vi "TLB Native Dynamic Events ver 0.25.vi"() -> ()   [LabVIEW 2018] (continued)
                }
              }
            }
          }
          frame 18 {
            # ">>> Motor control cluster >>>"
            # ">>> yStepper command>>>"
            # ">> Manual override >>"
            n401 = Equal?(x=w1065, y=u8 60) -> (x = y?=w1063:bool)
            n402 = Dequeue Element(queue=w1075, timeout in ms (-1)=w1074, error in (no error)=w1073) -> (element=w1072:T8)  [unwired: 3 out]
            n403 = case shown="\"Start Task 1\", Default" w1072 {
              tunnel: [w1084 State_Type_Definitions,_for_0.26g_versions_and_later_2."True Stop" ("Enum")] -> w1077
              tunnel: [w1087 w1104] -> w1070
              tunnel: [State_Type_Definitions,_for_0.26g_versions_and_later_2."Idle" ("Enum") State_Type_Definitions,_for_0.26g_versions_and_later_2."Shutdown" ("Enum")] -> w1069
              tunnel: w1071 -> [w1078 _]
              tunnel: w1076 -> [w1083 w1101]
              tunnel: w1063 -> [w1082 _]
              frame "Start Task 1", Default {
                # ">> Is time up? >>"
                # "Determines if object is in range to pick up"
                # ">> Manual override >>"
                n404 = case shown="True" w1082 {
                  tunnel: [w1091 w1097] -> w1087
                  tunnel: w1083 -> [w1089 w1095]
                  frame False {
                    n405 = for {
                      tunnel: string[] ["Z STEPPER CAM HEIGHT", "READ STEPPER VALUES"] ("element") -> [w1092] mode=indexing
                      shift-right: [w1094] -> w1091
                      shift-left: w1089 -> [w1093]
                      n406 = Enqueue Element(queue=w1093, element=w1092) -> (queue out=w1094:refnum<queue>)  [unwired: 2 in, 2 out]
                    }
                  }
                  frame True {
                    n407 = for {
                      shift-right: [w1099] -> w1097
                      shift-left: w1095 -> [w1100]
                      tunnel: string[] ["SET TIMER 5", "", ""] -> [w1098] mode=indexing
                      n408 = Enqueue Element(queue=w1100, element=w1098) -> (queue out=w1099:refnum<queue>)  [unwired: 2 in, 2 out]
                    }
                  }
                }
                n409 = Or(x=w1082, y=w1078) -> (x .or. y?=w1085:bool)
                n410 = Select(t=State_Type_Definitions,_for_0.26g_versions_and_later_2."True Stop" ("Enum"), s=w1078, f=State_Type_Definitions,_for_0.26g_versions_and_later_2."Task 5D" ("Enum")) -> (s? t:f=w1080:T16)
                n411 = Select(t=w1080, s=w1085, f=State_Type_Definitions,_for_0.26g_versions_and_later_2."Task 5C" ("Enum")) -> (s? t:f=w1084:T16)
              }
              frame "Exit" {
                n412 = for {
                  shift-right: [w1107] -> w1104
                  shift-left: w1101 -> [w1108]
                  tunnel: string[] ["STOP", "RESET ENCODERS", "RESET YAW", "ARDUINO MODE 0"] -> [w1106] mode=indexing
                  n413 = Enqueue Element(queue=w1108, element=w1106) -> (queue out=w1107:refnum<queue>)  [unwired: 2 in, 2 out]
                }
              }
            }
          }
          frame 19 {
            # ">>> yStepper command>>>"
            n414 = Dequeue Element(queue=w1116, timeout in ms (-1)=w1115, error in (no error)=w1114) -> (element=w1113:T8)  [unwired: 3 out]
            n415 = case shown="\"Start Task 1\", Default" w1113 {
              tunnel: [w1128 State_Type_Definitions,_for_0.26g_versions_and_later_2."True Stop" ("Enum")] -> w1120
              tunnel: [w1131 w1148] -> w1119
              tunnel: [State_Type_Definitions,_for_0.26g_versions_and_later_2."Idle" ("Enum") State_Type_Definitions,_for_0.26g_versions_and_later_2."Shutdown" ("Enum")] -> w1121
              tunnel: w1117 -> [w1127 _]
              tunnel: w1118 -> [w1123 w1145]
              tunnel: w1111 -> [w1122 _]
              frame "Start Task 1", Default {
                # ">> T: Breaks out of state loop; F: Stays in loop>>"
                # ">> Manual override >>"
                # ">> Checks if time is up>>"
                # "Stays in Task 5D until the object is detected"
                # "T: Go back to idle, F: Continue with task\""
                # ">> Manual override >>"
                n416 = case shown="False" w1122 {
                  tunnel: [w1135 w1141] -> w1131
                  tunnel: w1123 -> [w1133 w1139]
                  frame False {
                    n417 = for {
                      tunnel: string[] ["START TIMER", "OPEN CLAW", ""] ("element") -> [w1136] mode=indexing
                      shift-right: [w1138] -> w1135
                      shift-left: w1133 -> [w1137]
                      n418 = Enqueue Element(queue=w1137, element=w1136) -> (queue out=w1138:refnum<queue>)  [unwired: 2 in, 2 out]
                    }
                  }
                  frame True {
                    n419 = for {
                      shift-right: [w1143] -> w1141
                      shift-left: w1139 -> [w1144]
                      tunnel: string[] ["CAM CLOSE", "", ""] -> [w1142] mode=indexing
                      n420 = Enqueue Element(queue=w1144, element=w1142) -> (queue out=w1143:refnum<queue>)  [unwired: 2 in, 2 out]
                    }
                  }
                }
                n421 = Or(x=w1122, y=w1127) -> (x .or. y?=w1129:bool)
                n422 = Select(t=State_Type_Definitions,_for_0.26g_versions_and_later_2."True Stop" ("Enum"), s=w1127, f=State_Type_Definitions,_for_0.26g_versions_and_later_2."True Stop" ("Enum")) -> (s? t:f=w1124:T16)
                n423 = Select(t=w1124, s=w1129, f=State_Type_Definitions,_for_0.26g_versions_and_later_2."Task 5D" ("Enum")) -> (s? t:f=w1128:T16)
              }
              frame "Exit" {
                n424 = for {
                  shift-right: [w1151] -> w1148
                  shift-left: w1145 -> [w1152]
                  tunnel: string[] ["STOP", "RESET ENCODERS", "RESET YAW", "ARDUINO MODE 0"] -> [w1150] mode=indexing
                  n425 = Enqueue Element(queue=w1152, element=w1150) -> (queue out=w1151:refnum<queue>)  [unwired: 2 in, 2 out]
                }
              }
            }
          }
          frame 20 {
            # ">>> yStepper command>>>"
            n426 = Dequeue Element(queue=w1166, timeout in ms (-1)=w1167, error in (no error)=w1168) -> (element=w1170:T8)  [unwired: 3 out]
            n427 = formula code="if (pos < 100)\ny = 41;\n\nelse if (pos >= 100 && pos <= 140)\ny = 30;\n\nelse if (pos >= 141 && pos <= 170)\ny = 25;\n\nelse if (pos >= 171 &&pos <= 180) \ny = 20;\n\nelse if (pos >= 181&& pos <= 200)\ny = 15;\n\nelse if (pos >= 201 && pos <= 230)\ny = 10;\n\nelse if (pos >= 231 && pos <= 320)\ny = 8;\n\nelse if (pos > 320)\ny = 0;"("pos"=w1158) -> ("y"=w1161:dbl)
            n428 = To Unsigned Byte Integer(number=w1161) -> (unsigned 8bit integer=w1156:u8)
            n429 = Equal?(x=w1157, y=w1156) -> (x = y?=w1155:bool)
            n430 = case shown="\"Start Task 1\", Default" w1170 {
              tunnel: [w1177 State_Type_Definitions,_for_0.26g_versions_and_later_2."True Stop" ("Enum")] -> w1164
              tunnel: [w1180 w1197] -> w1162
              tunnel: [State_Type_Definitions,_for_0.26g_versions_and_later_2."Idle" ("Enum") State_Type_Definitions,_for_0.26g_versions_and_later_2."Shutdown" ("Enum")] -> w1163
              tunnel: w1169 -> [w1176 _]
              tunnel: w1165 -> [w1172 w1194]
              tunnel: w1155 -> [w1171 _]
              frame "Start Task 1", Default {
                # ">> T: Breaks out of state loop; F: Stays in loop>>"
                # ">> Manual override >>"
                # ">> Checks if time is up>>"
                # "Stays in Task 5D until the object is detected"
                # "T: Go back to idle, F: Continue with task\""
                # ">> Manual override >>"
                n431 = case shown="False" w1171 {
                  tunnel: [w1184 w1190] -> w1180
                  tunnel: w1172 -> [w1182 w1188]
                  frame False {
                    n432 = for {
                      tunnel: string[] ["READ STEPPER VALUES", "Y STEPPER CONTROL", ""] ("element") -> [w1185] mode=indexing
                      shift-right: [w1187] -> w1184
                      shift-left: w1182 -> [w1186]
                      n433 = Enqueue Element(queue=w1186, element=w1185) -> (queue out=w1187:refnum<queue>)  [unwired: 2 in, 2 out]
                    }
                  }
                  frame True {
                    n434 = for {
                      shift-right: [w1192] -> w1190
                      shift-left: w1188 -> [w1193]
                      tunnel: string[] ["CAM CLOSE", "DISPOSE BUFFERS", ""] -> [w1191] mode=indexing
                      n435 = Enqueue Element(queue=w1193, element=w1191) -> (queue out=w1192:refnum<queue>)  [unwired: 2 in, 2 out]
                    }
                  }
                }
                n436 = Or(x=w1171, y=w1176) -> (x .or. y?=w1178:bool)
                n437 = Select(t=State_Type_Definitions,_for_0.26g_versions_and_later_2."True Stop" ("Enum"), s=w1176, f=State_Type_Definitions,_for_0.26g_versions_and_later_2."Task 5F: ARM GRAB HEIGHT" ("Enum")) -> (s? t:f=w1173:T16)
                n438 = Select(t=w1173, s=w1178, f=State_Type_Definitions,_for_0.26g_versions_and_later_2."Task 5E: POSITION ARM" ("Enum")) -> (s? t:f=w1177:T16)
              }
              frame "Exit" {
                n439 = for {
                  shift-right: [w1200] -> w1197
                  shift-left: w1194 -> [w1201]
                  tunnel: string[] ["STOP", "RESET ENCODERS", "RESET YAW", "ARDUINO MODE 0"] -> [w1199] mode=indexing
                  n440 = Enqueue Element(queue=w1201, element=w1199) -> (queue out=w1200:refnum<queue>)  [unwired: 2 in, 2 out]
                }
              }
            }
            n441 = Bundle By Name(cluster=w1160, "yStepper desired"=w1156) -> (w1159:T18)
          }
          frame 21 {
            # ">>> Motor control cluster >>>"
            # ">>> yStepper command>>>"
            # ">> Manual override >>"
            n442 = Dequeue Element(queue=w1212, timeout in ms (-1)=w1211, error in (no error)=w1213) -> (element=w1210:T8)  [unwired: 3 out]
            n443 = Equal?(x=w1209, y=u8 1) -> (x = y?=w1207:bool)
            n444 = case shown="\"Start Task 1\", Default" w1210 {
              tunnel: [w1223 State_Type_Definitions,_for_0.26g_versions_and_later_2."True Stop" ("Enum")] -> w1214
              tunnel: [w1226 w1243] -> w1215
              tunnel: [State_Type_Definitions,_for_0.26g_versions_and_later_2."Idle" ("Enum") State_Type_Definitions,_for_0.26g_versions_and_later_2."Shutdown" ("Enum")] -> w1216
              tunnel: w1207 -> [w1222 _]
              tunnel: w1206 -> [w1221 _]
              tunnel: w1205 -> [w1217 w1240]
              frame "Start Task 1", Default {
                # "Stays in Task 5F until stepper reaches desired \nheight"
                # "T: Go back to idle, F: Continue with task\""
                # ">> Manual override >>"
                n445 = case shown="True" w1222 {
                  tunnel: [w1230 w1236] -> w1226
                  tunnel: w1217 -> [w1228 w1234]
                  frame False {
                    n446 = for {
                      tunnel: string[] ["Z STEPPER GRAB HEIGHT", "READ STEPPER VALUES"] ("element") -> [w1231] mode=indexing
                      shift-right: [w1233] -> w1230
                      shift-left: w1228 -> [w1232]
                      n447 = Enqueue Element(queue=w1232, element=w1231) -> (queue out=w1233:refnum<queue>)  [unwired: 2 in, 2 out]
                    }
                  }
                  frame True {
                    n448 = for {
                      shift-right: [w1238] -> w1236
                      shift-left: w1234 -> [w1239]
                      tunnel: string[] ["SET TIMER 5", "CLOSE CLAW", ""] -> [w1237] mode=indexing
                      n449 = Enqueue Element(queue=w1239, element=w1237) -> (queue out=w1238:refnum<queue>)  [unwired: 2 in, 2 out]
                    }
                  }
                }
                n450 = Or(x=w1222, y=w1221) -> (x .or. y?=w1224:bool)
                n451 = Select(t=State_Type_Definitions,_for_0.26g_versions_and_later_2."True Stop" ("Enum"), s=w1221, f=State_Type_Definitions,_for_0.26g_versions_and_later_2."Task 5G: CLOSE CLAW" ("Enum")) -> (s? t:f=w1218:T16)
                n452 = Select(t=w1218, s=w1224, f=State_Type_Definitions,_for_0.26g_versions_and_later_2."Task 5F: ARM GRAB HEIGHT" ("Enum")) -> (s? t:f=w1223:T16)
              }
              frame "Exit" {
                n453 = for {
                  shift-right: [w1246] -> w1243
                  shift-left: w1240 -> [w1247]
                  tunnel: string[] ["STOP", "RESET ENCODERS", "RESET YAW", "ARDUINO MODE 0"] -> [w1245] mode=indexing
                  n454 = Enqueue Element(queue=w1247, element=w1245) -> (queue out=w1246:refnum<queue>)  [unwired: 2 in, 2 out]
                }
              }
            }
          }
          frame 22 {
            # ">>> yStepper command>>>"
            # ">> Manual override >>"
            n455 = Dequeue Element(queue=w1258, timeout in ms (-1)=w1257, error in (no error)=w1256) -> (element=w1255:T8)  [unwired: 3 out]
            n456 = case shown="\"Start Task 1\", Default" w1255 {
              tunnel: [w1267 State_Type_Definitions,_for_0.26g_versions_and_later_2."True Stop" ("Enum")] -> w1260
              tunnel: [w1270 w1287] -> w1253
              tunnel: [State_Type_Definitions,_for_0.26g_versions_and_later_2."Idle" ("Enum") State_Type_Definitions,_for_0.26g_versions_and_later_2."Shutdown" ("Enum")] -> w1252
              tunnel: w1254 -> [w1261 _]
              tunnel: w1259 -> [w1266 w1284]
              tunnel: w1250 -> [w1265 _]
              frame "Start Task 1", Default {
                # ">> Is time up? >>"
                # "Determines if object is in range to pick up"
                # ">> Manual override >>"
                n457 = case shown="True" w1265 {
                  tunnel: [w1274 w1280] -> w1270
                  tunnel: w1266 -> [w1272 w1278]
                  frame False {
                    n458 = for {
                      tunnel: string[] ["CLOSE CLAW", "START TIMER"] ("element") -> [w1275] mode=indexing
                      shift-right: [w1277] -> w1274
                      shift-left: w1272 -> [w1276]
                      n459 = Enqueue Element(queue=w1276, element=w1275) -> (queue out=w1277:refnum<queue>)  [unwired: 2 in, 2 out]
                    }
                  }
                  frame True {
                    n460 = for {
                      shift-right: [w1282] -> w1280
                      shift-left: w1278 -> [w1283]
                      tunnel: string[] ["READ STEPPER VALUES", "", ""] -> [w1281] mode=indexing
                      n461 = Enqueue Element(queue=w1283, element=w1281) -> (queue out=w1282:refnum<queue>)  [unwired: 2 in, 2 out]
                    }
                  }
                }
                n462 = Or(x=w1265, y=w1261) -> (x .or. y?=w1268:bool)
                n463 = Select(t=State_Type_Definitions,_for_0.26g_versions_and_later_2."True Stop" ("Enum"), s=w1261, f=State_Type_Definitions,_for_0.26g_versions_and_later_2."Task 5H: RAISE ARM" ("Enum")) -> (s? t:f=w1263:T16)
                n464 = Select(t=w1263, s=w1268, f=State_Type_Definitions,_for_0.26g_versions_and_later_2."Task 5G: CLOSE CLAW" ("Enum")) -> (s? t:f=w1267:T16)
              }
              frame "Exit" {
                n465 = for {
                  shift-right: [w1290] -> w1287
                  shift-left: w1284 -> [w1291]
                  tunnel: string[] ["STOP", "RESET ENCODERS", "RESET YAW", "ARDUINO MODE 0"] -> [w1289] mode=indexing
                  n466 = Enqueue Element(queue=w1291, element=w1289) -> (queue out=w1290:refnum<queue>)  [unwired: 2 in, 2 out]
                }
              }
            }
          }
          frame 23 {
            # ">>> yStepper command>>>"
            # ">> Manual override >>"
            n467 = Dequeue Element(queue=w1302, timeout in ms (-1)=w1301, error in (no error)=w1303) -> (element=w1300:T8)  [unwired: 3 out]
            n468 = Equal?(x=w1299, y=u8 60) -> (x = y?=w1297:bool)
            n469 = case shown="\"Start Task 1\", Default" w1300 {
              tunnel: [w1313 State_Type_Definitions,_for_0.26g_versions_and_later_2."True Stop" ("Enum")] -> w1304
              tunnel: [w1316 w1333] -> w1305
              tunnel: [State_Type_Definitions,_for_0.26g_versions_and_later_2."Idle" ("Enum") State_Type_Definitions,_for_0.26g_versions_and_later_2."Shutdown" ("Enum")] -> w1306
              tunnel: w1297 -> [w1312 _]
              tunnel: w1296 -> [w1311 _]
              tunnel: w1295 -> [w1307 w1330]
              frame "Start Task 1", Default {
                # "Stays in Task 5_A until stepper reaches desired \nheight"
                # "T: Go back to idle, F: Continue with task\""
                # ">> Manual override >>"
                n470 = case shown="False" w1312 {
                  tunnel: [w1320 w1326] -> w1316
                  tunnel: w1307 -> [w1318 w1324]
                  frame False {
                    n471 = for {
                      tunnel: string[] ["Z STEPPER CAM HEIGHT", "READ STEPPER VALUES"] ("element") -> [w1321] mode=indexing
                      shift-right: [w1323] -> w1320
                      shift-left: w1318 -> [w1322]
                      n472 = Enqueue Element(queue=w1322, element=w1321) -> (queue out=w1323:refnum<queue>)  [unwired: 2 in, 2 out]
                    }
                  }
                  frame True {
                    n473 = for {
                      shift-right: [w1328] -> w1326
                      shift-left: w1324 -> [w1329]
                      tunnel: string[] ["ARDUINO - ULTRASONIC", "READ ULTRASONIC", ""] -> [w1327] mode=indexing
                      n474 = Enqueue Element(queue=w1329, element=w1327) -> (queue out=w1328:refnum<queue>)  [unwired: 2 in, 2 out]
                    }
                  }
                }
                n475 = Or(x=w1312, y=w1311) -> (x .or. y?=w1314:bool)
                n476 = Select(t=State_Type_Definitions,_for_0.26g_versions_and_later_2."True Stop" ("Enum"), s=w1311, f=State_Type_Definitions,_for_0.26g_versions_and_later_2."True Stop" ("Enum")) -> (s? t:f=w1308:T16)
                n477 = Select(t=w1308, s=w1314, f=State_Type_Definitions,_for_0.26g_versions_and_later_2."Task 5H: RAISE ARM" ("Enum")) -> (s? t:f=w1313:T16)
              }
              frame "Exit" {
                n478 = for {
                  shift-right: [w1336] -> w1333
                  shift-left: w1330 -> [w1337]
                  tunnel: string[] ["STOP", "RESET ENCODERS", "RESET YAW", "ARDUINO MODE 0"] -> [w1335] mode=indexing
                  n479 = Enqueue Element(queue=w1337, element=w1335) -> (queue out=w1336:refnum<queue>)  [unwired: 2 in, 2 out]
                }
              }
            }
          }
          frame 24 {
            # ">>> yStepper command>>>"
            n480 = Dequeue Element(queue=w1347, timeout in ms (-1)=w1346, error in (no error)=w1345) -> (element=w1352:T8)  [unwired: 3 out]
            n481 = Equal?(x=w1343, y=u8 60) -> (x = y?=w1342:bool)
            n482 = case shown="\"Start Task 1\", Default" w1352 {
              tunnel: [w1359 State_Type_Definitions,_for_0.26g_versions_and_later_2."True Stop" ("Enum")] -> w1350
              tunnel: [w1358 w1376] -> w1349
              tunnel: [State_Type_Definitions,_for_0.26g_versions_and_later_2."Idle" ("Enum") State_Type_Definitions,_for_0.26g_versions_and_later_2."Shutdown" ("Enum")] -> w1351
              tunnel: w1348 -> [w1354 _]
              tunnel: w1344 -> [w1356 _]
              tunnel: w1342 -> [w1353 _]
              frame "Start Task 1", Default {
                n483 = case shown="False" w1353 {
                  tunnel: [w1364 w1370] -> w1358
                  tunnel: w1356 -> [w1362 w1368]
                  frame False {
                    n484 = for {
                      tunnel: string[] ["Z STEPPER CAM HEIGHT", "READ STEPPER VALUES"] ("element") -> [w1365] mode=indexing
                      shift-right: [w1367] -> w1364
                      shift-left: w1362 -> [w1366]
                      n485 = Enqueue Element(queue=w1366, element=w1365) -> (queue out=w1367:refnum<queue>)  [unwired: 2 in, 2 out]
                    }
                  }
                  frame True {
                    n486 = for {
                      shift-right: [w1372] -> w1370
                      shift-left: w1368 -> [w1373]
                      tunnel: string[] ["CAM ACQ", "OPEN LOG CAM"] -> [w1371] mode=indexing
                      n487 = Enqueue Element(queue=w1373, element=w1371) -> (queue out=w1372:refnum<queue>)  [unwired: 2 in, 2 out]
                    }
                  }
                }
                n488 = Or(x=w1353, y=w1354) -> (x .or. y?=w1355:bool)
                n489 = Select(t=State_Type_Definitions,_for_0.26g_versions_and_later_2."Task 6_B" ("Enum"), s=w1355, f=State_Type_Definitions,_for_0.26g_versions_and_later_2."Task 6_A" ("Enum")) -> (s? t:f=w1359:T16)
              }
              frame "Exit" {
                n490 = for {
                  shift-right: [w1379] -> w1376
                  shift-left: _ -> [w1380]
                  tunnel: string[] ["STOP", "RESET ENCODERS", "RESET YAW", "ARDUINO MODE 0"] -> [w1378] mode=indexing
                  n491 = Enqueue Element(queue=w1380, element=w1378) -> (queue out=w1379:refnum<queue>)  [unwired: 2 in, 2 out]
                }
              }
            }
          }
          frame 25 {
            # ">>> yStepper command>>>"
            n492 = Dequeue Element(queue=w1392, timeout in ms (-1)=w1390, error in (no error)=w1391) -> (element=w1389:T8)  [unwired: 3 out]
            n493 = case shown="\"Start Task 1\", Default" w1389 {
              tunnel: [w1399 State_Type_Definitions,_for_0.26g_versions_and_later_2."True Stop" ("Enum")] -> w1385
              tunnel: [w1398 w1417] -> w1393
              tunnel: [State_Type_Definitions,_for_0.26g_versions_and_later_2."Idle" ("Enum") State_Type_Definitions,_for_0.26g_versions_and_later_2."Shutdown" ("Enum")] -> w1386
              tunnel: w1388 -> [w1394 _]
              tunnel: w1387 -> [w1396 _]
              tunnel: w1384 -> [w1395 w1414]
              frame "Start Task 1", Default {
                # ">> Manual override >>"
                n494 = case shown="False" w1396 {
                  tunnel: [w1404 w1410] -> w1398
                  tunnel: w1395 -> [w1403 w1408]
                  frame False {
                    n495 = for {
                      shift-right: [w1407] -> w1404
                      shift-left: w1403 -> [w1406]
                      tunnel: string[] ["CAM ACQ", "PROCESS IMAGE", "OPEN CLAW"] -> [w1405] mode=indexing
                      n496 = Enqueue Element(queue=w1406, element=w1405) -> (queue out=w1407:refnum<queue>)  [unwired: 2 in, 2 out]
                    }
                  }
                  frame True {
                    n497 = for {
                      shift-right: [w1412] -> w1410
                      shift-left: w1408 -> [w1413]
                      tunnel: string[] ["CAM ACQ", "PROCESS IMAGE", "CLOSE CLAW"] -> [w1411] mode=indexing
                      n498 = Enqueue Element(queue=w1413, element=w1411) -> (queue out=w1412:refnum<queue>)  [unwired: 2 in, 2 out]
                    }
                  }
                }
                n499 = Select(t=State_Type_Definitions,_for_0.26g_versions_and_later_2."True Stop" ("Enum"), s=w1394, f=State_Type_Definitions,_for_0.26g_versions_and_later_2."Task 6_B" ("Enum")) -> (s? t:f=w1399:T16)
              }
              frame "Exit" {
                # ">> State after true stop >>"
                # ">> Goes to true stop >>"
                n500 = for {
                  shift-right: [w1420] -> w1417
                  shift-left: w1414 -> [w1421]
                  tunnel: string[] ["STOP", "RESET ENCODERS", "RESET YAW", ""] -> [w1419] mode=indexing
                  n501 = Enqueue Element(queue=w1421, element=w1419) -> (queue out=w1420:refnum<queue>)  [unwired: 2 in, 2 out]
                }
              }
            }
          }
          frame 26 {
          }
          frame 27 {
            # ">>> Motor control cluster >>>"
            # ">>> yStepper command>>>"
            # ">> Manual override >>"
            n502 = Dequeue Element(queue=w1438, timeout in ms (-1)=w1437, error in (no error)=w1439) -> (element=w1436:T8)  [unwired: 3 out]
            n503 = Equal?(x=w1435, y=u8 60) -> (x = y?=w1433:bool)
            n504 = case shown="\"Start Task 1\", Default" w1436 {
              tunnel: [w1449 State_Type_Definitions,_for_0.26g_versions_and_later_2."True Stop" ("Enum")] -> w1440
              tunnel: [w1452 w1469] -> w1441
              tunnel: [State_Type_Definitions,_for_0.26g_versions_and_later_2."Idle" ("Enum") State_Type_Definitions,_for_0.26g_versions_and_later_2."Shutdown" ("Enum")] -> w1442
              tunnel: w1433 -> [w1448 _]
              tunnel: w1432 -> [w1447 _]
              tunnel: w1431 -> [w1443 w1466]
              frame "Start Task 1", Default {
                # "Stays in Task 5_A until stepper reaches desired \nheight"
                # "T: Go back to idle, F: Continue with task\""
                # ">> Manual override >>"
                n505 = case shown="False" w1448 {
                  tunnel: [w1456 w1462] -> w1452
                  tunnel: w1443 -> [w1454 w1460]
                  frame False {
                    n506 = for {
                      tunnel: string[] ["Z STEPPER CAM HEIGHT", "READ STEPPER VALUES"] ("element") -> [w1457] mode=indexing
                      shift-right: [w1459] -> w1456
                      shift-left: w1454 -> [w1458]
                      n507 = Enqueue Element(queue=w1458, element=w1457) -> (queue out=w1459:refnum<queue>)  [unwired: 2 in, 2 out]
                    }
                  }
                  frame True {
                    n508 = for {
                      shift-right: [w1464] -> w1462
                      shift-left: w1460 -> [w1465]
                      tunnel: string[] ["ARDUINO - ULTRASONIC", "READ ULTRASONIC", ""] -> [w1463] mode=indexing
                      n509 = Enqueue Element(queue=w1465, element=w1463) -> (queue out=w1464:refnum<queue>)  [unwired: 2 in, 2 out]
                    }
                  }
                }
                n510 = Or(x=w1448, y=w1447) -> (x .or. y?=w1450:bool)
                n511 = Select(t=State_Type_Definitions,_for_0.26g_versions_and_later_2."True Stop" ("Enum"), s=w1447, f=State_Type_Definitions,_for_0.26g_versions_and_later_2."Task 8B: MOVE TO BOX" ("Enum")) -> (s? t:f=w1444:T16)
                n512 = Select(t=w1444, s=w1450, f=State_Type_Definitions,_for_0.26g_versions_and_later_2."Task 8A: RAISE ARM" ("Enum")) -> (s? t:f=w1449:T16)
              }
              frame "Exit" {
                n513 = for {
                  shift-right: [w1472] -> w1469
                  shift-left: w1466 -> [w1473]
                  tunnel: string[] ["STOP", "RESET ENCODERS", "RESET YAW", "ARDUINO MODE 0"] -> [w1471] mode=indexing
                  n514 = Enqueue Element(queue=w1473, element=w1471) -> (queue out=w1472:refnum<queue>)  [unwired: 2 in, 2 out]
                }
              }
            }
          }
          frame 28 {
            w1481 = u8 15 ("y")
            # ">>> yStepper command>>>"
            n515 = Less?(x=w1478, y=w1481) -> (x < y?=w1479:bool)
            n516 = Dequeue Element(queue=w1485, timeout in ms (-1)=w1484, error in (no error)=w1486) -> (element=w1483:T8)  [unwired: 3 out]
            n517 = Less?(x=w1477, y=w1481) -> (x < y?=w1480:bool)
            n518 = And(x=w1480, y=w1479) -> (x .and. y?=w1476:bool)
            n519 = case shown="\"Start Task 1\", Default" w1483 {
              tunnel: [w1498 State_Type_Definitions,_for_0.26g_versions_and_later_2."True Stop" ("Enum")] -> w1488
              tunnel: [w1501 w1518] -> w1487
              tunnel: [State_Type_Definitions,_for_0.26g_versions_and_later_2."Idle" ("Enum") State_Type_Definitions,_for_0.26g_versions_and_later_2."Shutdown" ("Enum")] -> w1489
              tunnel: w1491 -> [w1497 _]
              tunnel: w1490 -> [w1493 w1515]
              tunnel: w1476 -> [w1492 _]
              frame "Start Task 1", Default {
                # "Stays in Task 5_B to capture image over 5 seconds"
                # "T: Go back to idle, F: Continue with task\""
                # ">> Manual override >>"
                n520 = case shown="True" w1492 {
                  tunnel: [w1505 w1511] -> w1501
                  tunnel: w1493 -> [w1503 w1509]
                  frame False {
                    n521 = for {
                      tunnel: string[] ["FORWARD", "READ ULTRASONIC", "READ NAVX"] ("element") -> [w1506] mode=indexing
                      shift-right: [w1508] -> w1505
                      shift-left: w1503 -> [w1507]
                      n522 = Enqueue Element(queue=w1507, element=w1506) -> (queue out=w1508:refnum<queue>)  [unwired: 2 in, 2 out]
                    }
                  }
                  frame True {
                    n523 = for {
                      shift-right: [w1513] -> w1511
                      shift-left: w1509 -> [w1514]
                      tunnel: string[] ["STOP", "RESET ENCODERS", "OPEN LOG CAM", "SET TIMER 2", "OPEN IMAQ REF"] -> [w1512] mode=indexing
                      n524 = Enqueue Element(queue=w1514, element=w1512) -> (queue out=w1513:refnum<queue>)  [unwired: 2 in, 2 out]
                    }
                  }
                }
                n525 = Or(x=w1492, y=w1497) -> (x .or. y?=w1499:bool)
                n526 = Select(t=State_Type_Definitions,_for_0.26g_versions_and_later_2."True Stop" ("Enum"), s=w1497, f=State_Type_Definitions,_for_0.26g_versions_and_later_2."Task 8C: CAM BURST" ("Enum")) -> (s? t:f=w1494:T16)
                n527 = Select(t=w1494, s=w1499, f=State_Type_Definitions,_for_0.26g_versions_and_later_2."Task 8B: MOVE TO BOX" ("Enum")) -> (s? t:f=w1498:T16)
              }
              frame "Exit" {
                n528 = for {
                  shift-right: [w1521] -> w1518
                  shift-left: w1515 -> [w1522]
                  tunnel: string[] ["STOP", "RESET ENCODERS", "RESET YAW", "ARDUINO MODE 0"] -> [w1520] mode=indexing
                  n529 = Enqueue Element(queue=w1522, element=w1520) -> (queue out=w1521:refnum<queue>)  [unwired: 2 in, 2 out]
                }
              }
            }
          }
          frame 29 {
            # ">>> Motor control cluster >>>"
            # ">>> yStepper command>>>"
            # ">> Manual override >>"
            n530 = Dequeue Element(queue=w1533, timeout in ms (-1)=w1532, error in (no error)=w1531) -> (element=w1530:T8)  [unwired: 3 out]
            n531 = case shown="\"Start Task 1\", Default" w1530 {
              tunnel: [w1542 State_Type_Definitions,_for_0.26g_versions_and_later_2."True Stop" ("Enum")] -> w1535
              tunnel: [w1545 w1562] -> w1528
              tunnel: [State_Type_Definitions,_for_0.26g_versions_and_later_2."Idle" ("Enum") State_Type_Definitions,_for_0.26g_versions_and_later_2."Shutdown" ("Enum")] -> w1527
              tunnel: w1529 -> [w1536 _]
              tunnel: w1534 -> [w1541 w1559]
              tunnel: w1525 -> [w1540 _]
              frame "Start Task 1", Default {
                # ">> Is time up? >>"
                # "Determines if object is in range to pick up"
                # ">> Manual override >>"
                n532 = case shown="True" w1540 {
                  tunnel: [w1549 w1555] -> w1545
                  tunnel: w1541 -> [w1547 w1553]
                  frame False {
                    n533 = for {
                      tunnel: string[] ["CAM ACQ", "START TIMER"] ("element") -> [w1550] mode=indexing
                      shift-right: [w1552] -> w1549
                      shift-left: w1547 -> [w1551]
                      n534 = Enqueue Element(queue=w1551, element=w1550) -> (queue out=w1552:refnum<queue>)  [unwired: 2 in, 2 out]
                    }
                  }
                  frame True {
                    n535 = for {
                      shift-right: [w1557] -> w1555
                      shift-left: w1553 -> [w1558]
                      tunnel: string[] ["CAM CLOSE", "PROCESS IMAGE", "SET TIMER 5"] -> [w1556] mode=indexing
                      n536 = Enqueue Element(queue=w1558, element=w1556) -> (queue out=w1557:refnum<queue>)  [unwired: 2 in, 2 out]
                    }
                  }
                }
                n537 = Or(x=w1540, y=w1536) -> (x .or. y?=w1543:bool)
                n538 = Select(t=State_Type_Definitions,_for_0.26g_versions_and_later_2."True Stop" ("Enum"), s=w1536, f=State_Type_Definitions,_for_0.26g_versions_and_later_2."Task 8D: PROCESS IMAGE" ("Enum")) -> (s? t:f=w1538:T16)
                n539 = Select(t=w1538, s=w1543, f=State_Type_Definitions,_for_0.26g_versions_and_later_2."Task 8C: CAM BURST" ("Enum")) -> (s? t:f=w1542:T16)
              }
              frame "Exit" {
                n540 = for {
                  shift-right: [w1565] -> w1562
                  shift-left: w1559 -> [w1566]
                  tunnel: string[] ["STOP", "RESET ENCODERS", "RESET YAW", "ARDUINO MODE 0"] -> [w1564] mode=indexing
                  n541 = Enqueue Element(queue=w1566, element=w1564) -> (queue out=w1565:refnum<queue>)  [unwired: 2 in, 2 out]
                }
              }
            }
          }
          frame 30 {
            # ">>> yStepper command>>>"
            n542 = Dequeue Element(queue=w1574, timeout in ms (-1)=w1573, error in (no error)=w1572) -> (element=w1571:T8)  [unwired: 3 out]
            n543 = case shown="\"Start Task 1\", Default" w1571 {
              tunnel: [w1586 State_Type_Definitions,_for_0.26g_versions_and_later_2."True Stop" ("Enum")] -> w1578
              tunnel: [w1589 w1606] -> w1577
              tunnel: [State_Type_Definitions,_for_0.26g_versions_and_later_2."Idle" ("Enum") State_Type_Definitions,_for_0.26g_versions_and_later_2."Shutdown" ("Enum")] -> w1579
              tunnel: w1575 -> [w1585 _]
              tunnel: w1576 -> [w1581 w1603]
              tunnel: w1569 -> [w1580 _]
              frame "Start Task 1", Default {
                # ">> T: Breaks out of state loop; F: Stays in loop>>"
                # ">> Manual override >>"
                # ">> Checks if time is up>>"
                # "Stays in Task 5D until the object is detected"
                # "T: Go back to idle, F: Continue with task\""
                # ">> Manual override >>"
                n544 = case shown="True" w1580 {
                  tunnel: [w1593 w1599] -> w1589
                  tunnel: w1581 -> [w1591 w1597]
                  frame False {
                    n545 = for {
                      tunnel: string[] ["START TIMER", "PROCESS IMAGE", ""] ("element") -> [w1594] mode=indexing
                      shift-right: [w1596] -> w1593
                      shift-left: w1591 -> [w1595]
                      n546 = Enqueue Element(queue=w1595, element=w1594) -> (queue out=w1596:refnum<queue>)  [unwired: 2 in, 2 out]
                    }
                  }
                  frame True {
                    n547 = for {
                      shift-right: [w1601] -> w1599
                      shift-left: w1597 -> [w1602]
                      tunnel: string[] ["RESET ENCODERS", "", ""] -> [w1600] mode=indexing
                      n548 = Enqueue Element(queue=w1602, element=w1600) -> (queue out=w1601:refnum<queue>)  [unwired: 2 in, 2 out]
                    }
                  }
                }
                n549 = Or(x=w1580, y=w1585) -> (x .or. y?=w1587:bool)
                n550 = Select(t=State_Type_Definitions,_for_0.26g_versions_and_later_2."True Stop" ("Enum"), s=w1585, f=State_Type_Definitions,_for_0.26g_versions_and_later_2."Task 8E: ROBOT ADJUST" ("Enum")) -> (s? t:f=w1582:T16)
                n551 = Select(t=w1582, s=w1587, f=State_Type_Definitions,_for_0.26g_versions_and_later_2."Task 8D: PROCESS IMAGE" ("Enum")) -> (s? t:f=w1586:T16)
              }
              frame "Exit" {
                n552 = for {
                  shift-right: [w1609] -> w1606
                  shift-left: w1603 -> [w1610]
                  tunnel: string[] ["STOP", "RESET ENCODERS", "RESET YAW", "ARDUINO MODE 0"] -> [w1608] mode=indexing
                  n553 = Enqueue Element(queue=w1610, element=w1608) -> (queue out=w1609:refnum<queue>)  [unwired: 2 in, 2 out]
                }
              }
            }
          }
          frame 31 {
            # ">>> Motor control cluster >>>"
            # ">>> yStepper command>>>"
            n554 = Dequeue Element(queue=w1627, timeout in ms (-1)=w1626, error in (no error)=w1625) -> (element=w1624:T8)  [unwired: 3 out]
            n555 = Subtract(x=w1622, y=300.0) -> (x-y=w1620:dbl)
            n556 = formula code="if (error <= -61&&error > -300){\ndistance = -15;\nxSpeed = -30;\n}\n\nelse if (error <= -51 && error >= -60){\ndistance = -10;\nxSpeed = -30;\n}\n\nelse if (error >= -50 && error <= 50){\ndistance = 0;\nxSpeed = 0;\n}\n\nelse if (error >= 51 && error <= 80){\ndistance = 10;\nxSpeed = 30;\n}\n\nelse if (error >= 81 && error <= 100){\ndistance = 15;\nxSpeed = 30;\n}\n\nelse if (error >= 101 && error <= 120){\ndistance = 20;\nxSpeed = 30;\n}\n\nelse if (error >= 121 && error < 300){\ndistance = 25;\nxSpeed = 30;\n}\n\nelse{\ndistance = 0;\nxSpeed = 0;\n}"("error"=w1620) -> ("distance"=w1615:dbl, "xSpeed"=w1617:dbl)
            n557 = formula code="if (target > 0){\nif (current  >= target)\noutput = 1;\n\nelse if (current != target)\noutput = 0;\n}\n\nelse if (target == 0){\nif (current == target)\noutput = 1;\n\nelse if (current != target)\noutput = 0;\n}\n\nelse if (target < 0){\nif (current <= target)\noutput = 1;\n\nelse if (current != target)\noutput = 0;\n}\n\nelse if (current != target)\noutput = 0;"("target"=w1615, "current"=w1616) -> ("output"=w1614:dbl)
            n558 = Bundle By Name(cluster=w1619, "xSpeed"=w1617) -> (w1618:T17)
            n559 = Equal?(x=w1614, y=1.0) -> (x = y?=w1612:bool)
            n560 = case shown="\"Start Task 1\", Default" w1624 {
              tunnel: [w1639 State_Type_Definitions,_for_0.26g_versions_and_later_2."True Stop" ("Enum")] -> w1631
              tunnel: [w1642 w1659] -> w1630
              tunnel: [State_Type_Definitions,_for_0.26g_versions_and_later_2."Idle" ("Enum") State_Type_Definitions,_for_0.26g_versions_and_later_2."Shutdown" ("Enum")] -> w1632
              tunnel: w1628 -> [w1638 _]
              tunnel: w1629 -> [w1634 w1656]
              tunnel: w1612 -> [w1633 _]
              frame "Start Task 1", Default {
                # ">> T: Breaks out of state loop; F: Stays in loop>>"
                # ">> Manual override >>"
                # ">> Checks if time is up>>"
                # "Stays in Task 5D until the object is detected"
                # "T: Go back to idle, F: Continue with task\""
                # ">> Manual override >>"
                n561 = case shown="True" w1633 {
                  tunnel: [w1646 w1652] -> w1642
                  tunnel: w1634 -> [w1644 w1650]
                  frame False {
                    n562 = for {
                      tunnel: string[] ["X AXIS - SLOW", "READ ENCODERS", "READ NAVX"] ("element") -> [w1647] mode=indexing
                      shift-right: [w1649] -> w1646
                      shift-left: w1644 -> [w1648]
                      n563 = Enqueue Element(queue=w1648, element=w1647) -> (queue out=w1649:refnum<queue>)  [unwired: 2 in, 2 out]
                    }
                  }
                  frame True {
                    n564 = for {
                      shift-right: [w1654] -> w1652
                      shift-left: w1650 -> [w1655]
                      tunnel: string[] ["SET TIMER 2", "STOP", "READ STEPPER VALUES", ""] -> [w1653] mode=indexing
                      n565 = Enqueue Element(queue=w1655, element=w1653) -> (queue out=w1654:refnum<queue>)  [unwired: 2 in, 2 out]
                    }
                  }
                }
                n566 = Or(x=w1633, y=w1638) -> (x .or. y?=w1640:bool)
                n567 = Select(t=State_Type_Definitions,_for_0.26g_versions_and_later_2."True Stop" ("Enum"), s=w1638, f=State_Type_Definitions,_for_0.26g_versions_and_later_2."Task 8H: ARM ADJUST" ("Enum")) -> (s? t:f=w1635:T16)
                n568 = Select(t=w1635, s=w1640, f=State_Type_Definitions,_for_0.26g_versions_and_later_2."Task 8E: ROBOT ADJUST" ("Enum")) -> (s? t:f=w1639:T16)
              }
              frame "Exit" {
                n569 = for {
                  shift-right: [w1662] -> w1659
                  shift-left: w1656 -> [w1663]
                  tunnel: string[] ["STOP", "RESET ENCODERS", "RESET YAW", "ARDUINO MODE 0"] -> [w1661] mode=indexing
                  n570 = Enqueue Element(queue=w1663, element=w1661) -> (queue out=w1662:refnum<queue>)  [unwired: 2 in, 2 out]
                }
              }
            }
          }
          frame 32 {
            # ">>> Motor control cluster >>>"
            # ">>> yStepper command>>>"
            # ">> Manual override >>"
            n571 = Dequeue Element(queue=w1674, timeout in ms (-1)=w1673, error in (no error)=w1672) -> (element=w1671:T8)  [unwired: 3 out]
            n572 = case shown="\"Start Task 1\", Default" w1671 {
              tunnel: [w1683 State_Type_Definitions,_for_0.26g_versions_and_later_2."True Stop" ("Enum")] -> w1676
              tunnel: [w1686 w1703] -> w1669
              tunnel: [State_Type_Definitions,_for_0.26g_versions_and_later_2."Idle" ("Enum") State_Type_Definitions,_for_0.26g_versions_and_later_2."Shutdown" ("Enum")] -> w1668
              tunnel: w1670 -> [w1677 _]
              tunnel: w1675 -> [w1682 w1700]
              tunnel: w1666 -> [w1681 _]
              frame "Start Task 1", Default {
                # ">> Is time up? >>"
                # "Determines if object is in range to pick up"
                # ">> Manual override >>"
                n573 = case shown="False" w1681 {
                  tunnel: [w1690 w1696] -> w1686
                  tunnel: w1682 -> [w1688 w1694]
                  frame False {
                    n574 = for {
                      tunnel: string[] ["CAM ACQ", "START TIMER"] ("element") -> [w1691] mode=indexing
                      shift-right: [w1693] -> w1690
                      shift-left: w1688 -> [w1692]
                      n575 = Enqueue Element(queue=w1692, element=w1691) -> (queue out=w1693:refnum<queue>)  [unwired: 2 in, 2 out]
                    }
                  }
                  frame True {
                    n576 = for {
                      shift-right: [w1698] -> w1696
                      shift-left: w1694 -> [w1699]
                      tunnel: string[] ["CAM CLOSE", "PROCESS IMAGE", "SET TIMER 3"] -> [w1697] mode=indexing
                      n577 = Enqueue Element(queue=w1699, element=w1697) -> (queue out=w1698:refnum<queue>)  [unwired: 2 in, 2 out]
                    }
                  }
                }
                n578 = Or(x=w1681, y=w1677) -> (x .or. y?=w1684:bool)
                n579 = Select(t=State_Type_Definitions,_for_0.26g_versions_and_later_2."True Stop" ("Enum"), s=w1677, f=State_Type_Definitions,_for_0.26g_versions_and_later_2."Task 8G: PROCESS IMAGE 2" ("Enum")) -> (s? t:f=w1679:T16)
                n580 = Select(t=w1679, s=w1684, f=State_Type_Definitions,_for_0.26g_versions_and_later_2."Task 8F: CAM BURST 2" ("Enum")) -> (s? t:f=w1683:T16)
              }
              frame "Exit" {
                n581 = for {
                  shift-right: [w1706] -> w1703
                  shift-left: w1700 -> [w1707]
                  tunnel: string[] ["STOP", "RESET ENCODERS", "RESET YAW", "ARDUINO MODE 0"] -> [w1705] mode=indexing
                  n582 = Enqueue Element(queue=w1707, element=w1705) -> (queue out=w1706:refnum<queue>)  [unwired: 2 in, 2 out]
                }
              }
            }
          }
          frame 33 {
            # ">>> yStepper command>>>"
            n583 = Dequeue Element(queue=w1715, timeout in ms (-1)=w1714, error in (no error)=w1713) -> (element=w1712:T8)  [unwired: 3 out]
            n584 = case shown="\"Start Task 1\", Default" w1712 {
              tunnel: [w1727 State_Type_Definitions,_for_0.26g_versions_and_later_2."True Stop" ("Enum")] -> w1719
              tunnel: [w1730 w1747] -> w1718
              tunnel: [State_Type_Definitions,_for_0.26g_versions_and_later_2."Idle" ("Enum") State_Type_Definitions,_for_0.26g_versions_and_later_2."Shutdown" ("Enum")] -> w1720
              tunnel: w1716 -> [w1726 _]
              tunnel: w1717 -> [w1722 w1744]
              tunnel: w1710 -> [w1721 _]
              frame "Start Task 1", Default {
                # ">> T: Breaks out of state loop; F: Stays in loop>>"
                # ">> Manual override >>"
                # ">> Checks if time is up>>"
                # "Stays in Task 5D until the object is detected"
                # "T: Go back to idle, F: Continue with task\""
                # ">> Manual override >>"
                n585 = case shown="False" w1721 {
                  tunnel: [w1734 w1740] -> w1730
                  tunnel: w1722 -> [w1732 w1738]
                  frame False {
                    n586 = for {
                      tunnel: string[] ["START TIMER", "PROCESS IMAGE", ""] ("element") -> [w1735] mode=indexing
                      shift-right: [w1737] -> w1734
                      shift-left: w1732 -> [w1736]
                      n587 = Enqueue Element(queue=w1736, element=w1735) -> (queue out=w1737:refnum<queue>)  [unwired: 2 in, 2 out]
                    }
                  }
                  frame True {
                    n588 = for {
                      shift-right: [w1742] -> w1740
                      shift-left: w1738 -> [w1743]
                      tunnel: string[] ["READ STEPPER VALUES", "Y STEPPER CONTROL", ""] -> [w1741] mode=indexing
                      n589 = Enqueue Element(queue=w1743, element=w1741) -> (queue out=w1742:refnum<queue>)  [unwired: 2 in, 2 out]
                    }
                  }
                }
                n590 = Or(x=w1721, y=w1726) -> (x .or. y?=w1728:bool)
                n591 = Select(t=State_Type_Definitions,_for_0.26g_versions_and_later_2."True Stop" ("Enum"), s=w1726, f=State_Type_Definitions,_for_0.26g_versions_and_later_2."Task 8H: ARM ADJUST" ("Enum")) -> (s? t:f=w1723:T16)